vi "Exercise2.2-FM Modulation Demo (Single Tone)-IQ.vi"() -> ()   [LabVIEW 2013]
uses:
  <vilib>/express/express analysis/Spectral/Block/exnSpectralBlock spectral measurements power poly.vi
  <vilib>/express/express analysis/Spectral/XNode/ExpressSpectralMeasurementsBlockNode.xnode
  <vilib>/addons/Modulation/Analog/MT Passband PLL.vi
  <vilib>/express/express analysis/Spectral/Block/exnSpectralBlock spectral measurements power DDT.vi
  <vilib>/addons/Modulation/niAMT.lvlib
  <vilib>/Analysis/NI_AALPro.lvlib
panel:
  in  "Mod. Freq.":dbl=2000.0 caption="Frequency"
  out "Estimated freq.":dbl
  in  "WAV SR":dbl=44100.0 caption="dt"
  in  "LPF Cut-Off":dbl=60000.0 caption="Lower Cut-Off"
  in  "SNR (dB)":dbl(slide)=30.0 caption="Standard deviation" scale=-20.0..100.0
  out "Recovered Signal":dynamicdata(graph)=[{"t0"=timestamp(0 s since 1904-01-01), "dt"=1e-06, "Y"=array[100000 elements], "attributes"=variant("NI_ChannelName"=variant(string "Sine (Derivative (dX/dt))"), "NI_ExpIsRelativeTime"=variant(bool TRUE), "NI_ExpStartTimeStamp"=variant(timestamp timestamp(3676385695.5098023 s since 1904-01-01)), "NI_ExpTimeStamp"=variant(timestamp timestamp(3676385695.5098023 s since 1904-01-01)), "NI_ExpXDimension"=variant(string "t"), "NI_OriginalChannelName"=variant(string "Sine"))}]
  out "Baseband":dynamicdata(graph)=[{"t0"=timestamp(0 s since 1904-01-01), "dt"=1e-06, "Y"=array[100000 elements], "attributes"=variant("NI_ChannelName"=variant(string "Sine"), "NI_ExpIsRelativeTime"=variant(bool TRUE), "NI_ExpStartTimeStamp"=variant(timestamp timestamp(3676385695.5098023 s since 1904-01-01)), "NI_ExpTimeStamp"=variant(timestamp timestamp(3676385695.5098023 s since 1904-01-01)), "NI_ExpXDimension"=variant(string "t"))}]
  out "FM Spectrum":dynamicdata(graph)=[{"t0"=timestamp(0 s since 1904-01-01), "dt"=10.0, "Y"=array[50000 elements], "attributes"=variant("NI_ChannelName"=variant(string "Sine (Power Spectrum)"), "NI_ExpIsRelativeTime"=variant(bool TRUE), "NI_ExpStartTimeStamp"=variant(timestamp timestamp(3676385695.5098023 s since 1904-01-01)), "NI_ExpTimeStamp"=variant(timestamp timestamp(3676385695.5098023 s since 1904-01-01)), "NI_ExpXDimension"=variant(string "f"), "NI_OriginalChannelName"=variant(string "Sine"))}]
  out "FM Wave":dynamicdata(graph)=[{"t0"=timestamp(0 s since 1904-01-01), "dt"=1e-06, "Y"=array[100000 elements], "attributes"=variant("NI_ChannelName"=variant(string "Sine"), "NI_ExpIsRelativeTime"=variant(bool TRUE), "NI_ExpStartTimeStamp"=variant(timestamp timestamp(3676385695.5098023 s since 1904-01-01)), "NI_ExpTimeStamp"=variant(timestamp timestamp(3676385695.5098023 s since 1904-01-01)), "NI_ExpXDimension"=variant(string "t"))}, {"t0"=timestamp(0 s since 1904-01-01), "dt"=1e-06, "Y"=array[100000 elements], "attributes"=variant("NI_ChannelName"=variant(string "Sine (Integral (Sum[Xdt]))"), "NI_ExpIsRelativeTime"=variant(bool TRUE), "NI_ExpStartTimeStamp"=variant(timestamp timestamp(3676385695.5098023 s since 1904-01-01)), "NI_ExpTimeStamp"=variant(timestamp timestamp(3676385695.5098023 s since 1904-01-01)), "NI_ExpXDimension"=variant(string "t"), "NI_OriginalChannelName"=variant(string "Sine"))}]
  in  "Carrier Amp.":dbl=1.0 caption="Amplitude"
  in  "stop":bool
  in  "Frequency Deviation":dbl(slide)=200.0 scale=0.0..75000.0
  in  "Carrier Freq.":dbl=100000.0 caption="Frequency"
  # "正交解调低通滤波器的截止频率不应设置为基带信号频率，WBFM调频之后带宽增加！"
  # "Frequency Modulation"
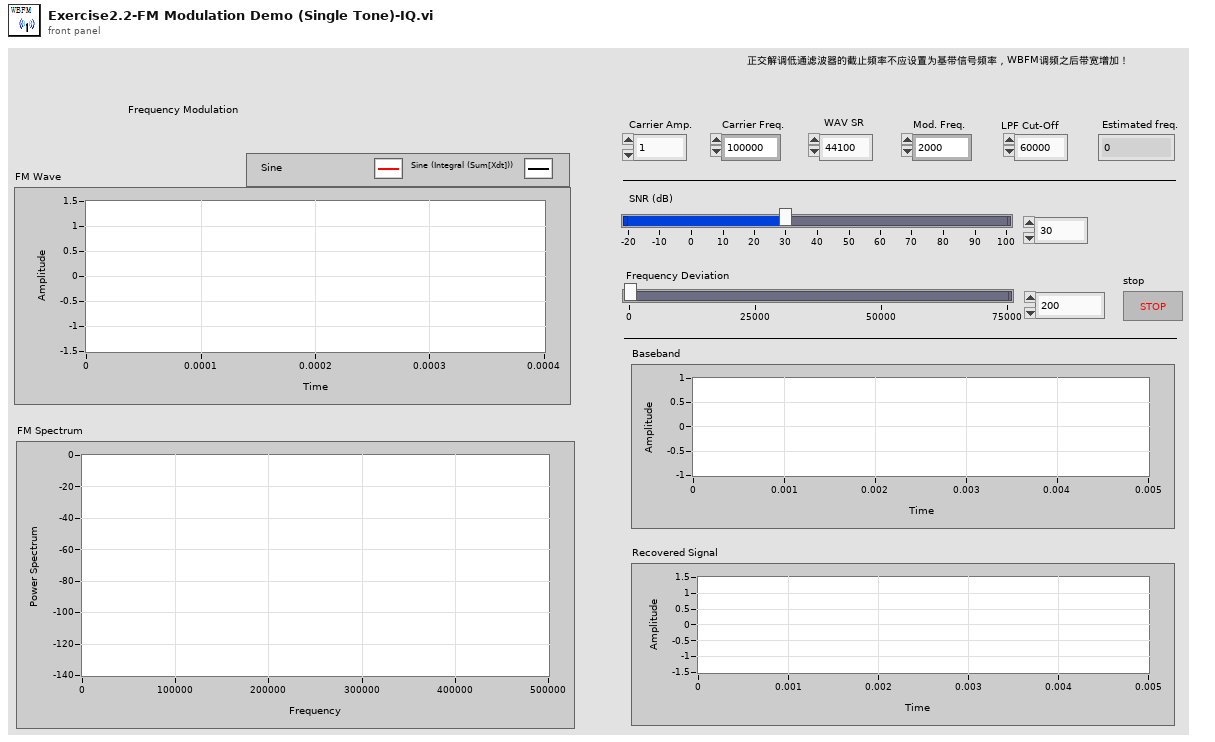
[diagram p1: front panel]
types:
  T1 = cluster{"averaging mode":u16, "weighting mode":u16, "number of averages":u32}
  T2 = cluster{"dB On (F)":bool, "unwrap phase (F)":bool, "convert to degree (F)":bool}
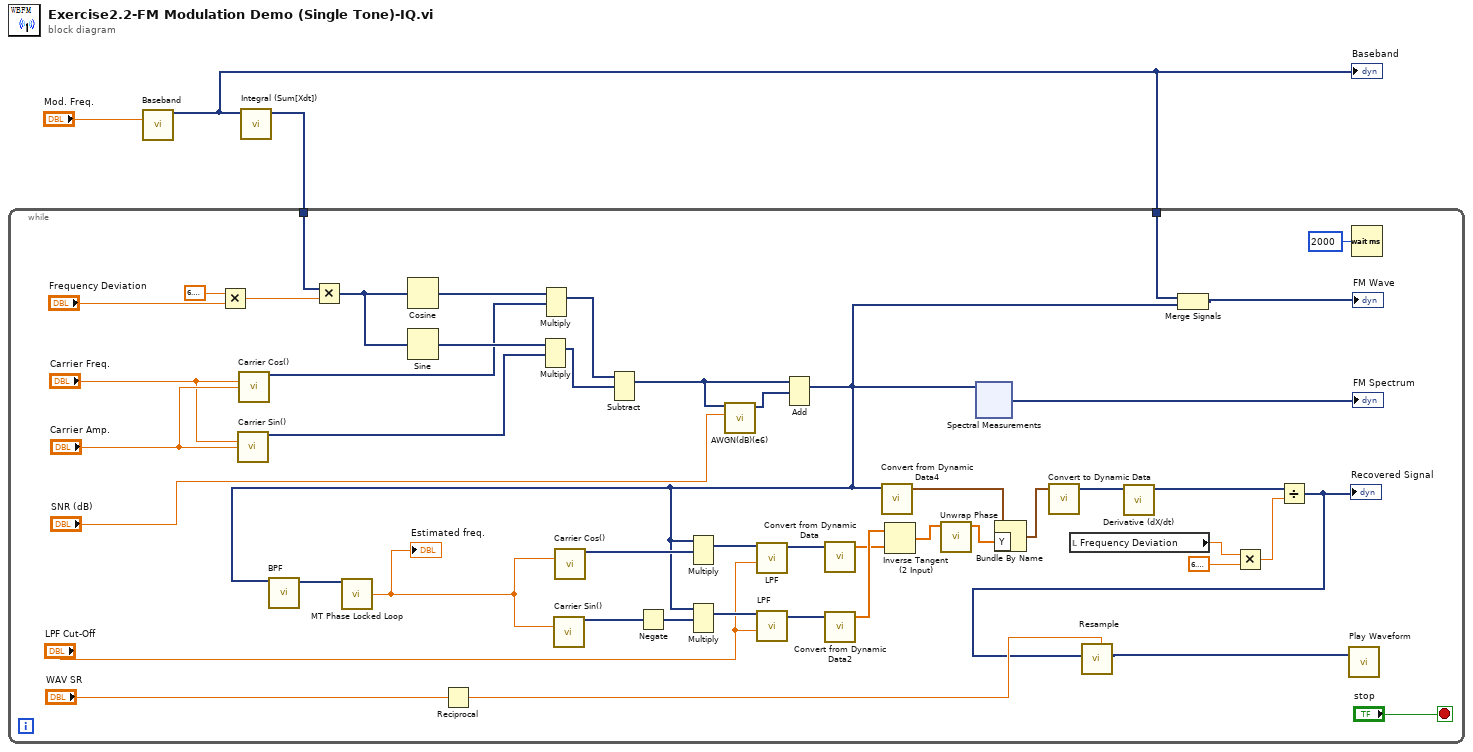
[diagram p0: block diagram]
diagram:
  n1 = call "Baseband"("Frequency"="Mod. Freq.") -> ("Sine"=w2:dynamicdata)  [unwired: 13 in, 1 out]
  "Baseband" <- w2
  n2 = call "Integral (Sum[Xdt])"("Signals"=w2) -> ("Result"=w3:dynamicdata)  [unwired: 5 in, 1 out]
  n3 = while {
    tunnel: w3 -> [w26]
    tunnel: w2 -> [w10]
    stop <- "stop" stop-if-true
    n4 = Multiply(x=6.283185307179586, y="Frequency Deviation") -> (x*y=w42:dbl)
    n5 = call "Carrier Sin()"("Frequency"="Carrier Freq.", "Amplitude"="Carrier Amp.") -> ("Sine"=w16:dynamicdata)  [unwired: 12 in, 1 out]
    n6 = call "Carrier Cos()"("Frequency"="Carrier Freq.", "Amplitude"="Carrier Amp.") -> ("Sine"=w17:dynamicdata)  [unwired: 12 in, 1 out]
    n7 = Multiply ("Multiplier")(x=w26, y=w42) -> (x*y=w38:dynamicdata)
    n8 = Cosine(x=w38) -> (cos(x)=w19:dynamicdata)
    n9 = Sine(x=w38) -> (sin(x)=w30:dynamicdata)
    n10 = Reciprocal(x="WAV SR") -> (1/x=w24:dbl)
    n11 = Multiply ("Multiplier")(1:w16, 2:w30) -> (0:w37:dynamicdata)  [unwired: 1 in, 1 out]
    n12 = Multiply ("Multiplier")(1:w17, 2:w19) -> (0:w25:dynamicdata)  [unwired: 1 in, 1 out]
    n13 = Subtract(1:w37, 2:w25) -> (0:w36:dynamicdata)  [unwired: 1 in, 1 out]
    n14 = call "AWGN(dB)(e6).vi"("AWGN (dB)"="SNR (dB)", "Dynamic Data"=w36) -> ("DC with Gaussian Noise"=w41:dynamicdata)  [unwired: 9 in]
    n15 = Add ("Adder")(1:w41, 2:w36) -> (0:w11:dynamicdata)  [unwired: 1 in, 1 out]
    n16 = call "BPF"("Signal"=w11) -> ("Filtered Signal"=w40:dynamicdata)  [unwired: 9 in, 1 out]
    n17 = call-poly <vilib>:"MT Phase Locked Loop.vi"("passband waveform"=w40) -> ("estimated carrier frequency (Hz)"=w39:dbl)  [unwired: 10 in, 4 out]
    "Estimated freq." <- w39
    n18 = call "Carrier Sin()"("Frequency"=w39) -> ("Sine"=w14:dynamicdata)  [unwired: 13 in, 1 out]
    n19 = call "Carrier Cos()"("Frequency"=w39) -> ("Sine"=w13:dynamicdata)  [unwired: 13 in, 1 out]
    n20 = Negate(x=w14) -> (-x=w32:dynamicdata)
    n21 = Multiply(1:w13, 2:w11) -> (0:w15:dynamicdata)  [unwired: 1 in, 1 out]
    n22 = Multiply(1:w32, 2:w11) -> (0:w34:dynamicdata)  [unwired: 1 in, 1 out]
    n23 = call "LPF"("Lower Cut-Off"="LPF Cut-Off", "Signal"=w15) -> ("Filtered Signal"=w12:dynamicdata)  [unwired: 8 in, 1 out]
    n24 = call "LPF"("Lower Cut-Off"="LPF Cut-Off", "Signal"=w34) -> ("Filtered Signal"=w31:dynamicdata)  [unwired: 8 in, 1 out]
    n25 = call "Convert from Dynamic Data"("Dynamic Data Type"=w12) -> ("Array"=w28:dbl[])  [unwired: 3 in]
    n26 = call "Convert from Dynamic Data2"("Dynamic Data Type"=w31) -> ("Array"=w29:dbl[])  [unwired: 3 in]
    n27 = call "Convert from Dynamic Data4"("Dynamic Data Type"=w11) -> ("Waveform"=w22:waveform(dbl))  [unwired: 3 in]
    n28 = Inverse Tangent (2 Input)(1:w28, 2:w29) -> (0:w27:dbl[])
    n29 = call <vilib>:"Unwrap Phase.vi"("Phase"=w27) -> ("Unwrapped Phase"=w23:dbl[])  [unwired: 9 in, 1 out]
    n30 = xnode "Spectral Measurements"("Signals"=w11) -> ("Power Spectrum"=→"FM Spectrum":dynamicdata)  [unwired: 1 in, 1 out]
    n31 = Bundle By Name(cluster=w22, "Y"=w23) -> (w21:waveform(dbl))
    n32 = call "Convert to Dynamic Data"("Waveform"=w21) -> ("Dynamic Data Type"=w20:dynamicdata)  [unwired: 3 in]
    n33 = local read "Frequency Deviation"() -> (w8:dbl)
    n34 = call "Derivative (dX/dt)"("Signals"=w20) -> ("Result"=w6:dynamicdata)  [unwired: 5 in, 1 out]
    n35 = Merge Signals(w10, w11) -> (→"FM Wave":dynamicdata)
    n36 = Multiply(x=w8, y=6.283185307179586) -> (x*y=w4:dbl)
    n37 = Divide(x=w6, y=w4) -> (x/y=w5:dynamicdata)
    "Recovered Signal" <- w5
    n38 = call "Resample"("dt"=w24, "Signals"=w5) -> ("Resampled Signals"=w9:dynamicdata)  [unwired: 7 in, 2 out]
    n39 = call "Play Waveform"("Data"=w9) -> ()  [unwired: 18 in, 1 out]
    n40 = Wait (ms)(milliseconds to wait=u32 2000) -> ()  [unwired: 1 out]
  }
